vi "CRYO_MASTER_FULL_RUN2.vi"() -> ()   [LabVIEW 2017] (continued)
  T23 = typedef "imagedata.ctl" = cluster{"image type":i32, "image depth":i32, "image":u8[], "mask":u8[], "colors":u32[], "Rectangle":cluster{"left":i16, "top":i16, "right":i16, "bottom":i16}}
  T24 = enum16{"open", "replace", "create", "open or create", "replace or create", "replace or create with confirmation"}
  T25 = cluster{"TimeArray":timestamp[], "DataArrayConv":dbl[]}[]
  T26 = cluster{"IndexArray":i64[], "TimeArray":timestamp[], "DataArrayRaw":dbl[][], "DataArrayConv":dbl[][], "LDArray":dbl[]}
  T27 = cluster{"InstName":string, "Active?":bool, "Status":enum16{"Intialized", "Ready", "Measuring", "Terminated"}, "Labels":string[], "LabelLD":string, "FileFormat":string[], "FileFormatLD":string, "ReadLeakDet?":bool}
  T28 = cluster{"AOUT Labels[0]":string, "AOUT Labels[1]":string, "AOUT Labels[2]":string, "AOUT Labels[3]":string, "AOUT Labels[4]":string, "AOUT Labels[5]":string, "AOUT Labels[6]":string, "AOUT Labels[7]":string, "AOUT Labels[8]":string}
  T29 = cluster{"TimeArray":timestamp[], "DataArrayConv":dbl[]}
  T30 = cluster{"TimeArray":timestamp[], "DataArrayConv (USB6218)":dbl[]}
  T31 = cluster{"TimeArray":timestamp[], "M.A. Array":dbl[]}
  T32 = cluster{"TimeArray":timestamp[], "M.A. Array":dbl[]}[]
  T33 = cluster{"TimeArray":timestamp[], "DataArray":dbl[]}
  T34 = enum16{"USB6210", "USB6218AI", "USB6218AO", "LSI218", "LSI336", "DMMs"}
diagram:
  w15 = TRUE ("create if not found? (T)")
  w19 = errorcluster {"status"=FALSE, "code"=0, "source"=""} ("error in (no error)")
  w4 = errorcluster {"status"=FALSE, "code"=0, "source"=""} ("error in (no error)")
  n1 = while {
    shift-right: [w42] -> _
    shift-left: dbl[] [] -> [w48]
    shift-right: [w45] -> _
    shift-left: timestamp[] [] -> [w47]
    i -> [w46]
    stop <- w49 stop-if-true
    n2 = Wait (ms)(milliseconds to wait=u32 225) -> ()  [unwired: 1 out]
    n3 = event shown="[6] \"OUTPUT (PWR)\", \"OUTPUT (PMC)\": Value Change" {
      selector: _ -> [_ _ _ _ _ _ _]
      dyn-events: _ -> [_ _ _ _ _ _ _]
      timeout: _ -> [_ _ _ _ _ _ _]
      tunnel: [_ TRUE _ _ _ _ _] -> w49
      tunnel: w46 -> [_ _ _ _ w130 _ _]
      tunnel: [_ _ _ _ w129 w213 _] -> w42
      tunnel: w48 -> [_ _ _ _ w126 w213 _]
      tunnel: [w51 w61 _ _ w128 w212 w216] -> w45
      tunnel: w47 -> [w51 w61 _ _ w127 w212 w216]
      tunnel: w46 -> [_ _ w67 w91 _ _ w217]
      tunnel: [_ _ _ _ w117 _ _] -> w41
      event Timeout {
        n4 = event-data() -> ()  [unwired: 1 in, 3 out]
      }
      event "Stop Button": Value Change {
        w52 = FALSE
        n5 = event-data() -> ()  [unwired: 1 in, 3 out]
        n6 = local read "error out (USB6210/6218 DOUT)"() -> (w60:errorcluster)
        n7 = local read "error out (USB6210/6218 AOUT)"() -> (w57:errorcluster)
        n8 = local read "DOUT task out"() -> (w56:refnum<k21>)
        n9 = local read "AO task out"() -> (w63:refnum<k21>)
        n10 = property on="OUTPUT\n(PWR)" class="Bool (strict)"("Value"=w52) -> ()  [unwired: 2 in, 2 out]
        n11 = property on="V2 (N.C.)" class="Bool (strict)"("Val(Sgnl)"=w52) -> ()  [unwired: 2 in, 2 out]
        n12 = property on="OUTPUT\n(PMC)" class="Bool (strict)"("Value"=w52) -> ()  [unwired: 2 in, 2 out]
        n13 = Build Array(w52, w52, w52, w52) -> (w59:bool[])
        n14 = Not(x=w52) -> (.not. x?=w53:bool)
        n15 = call <vilib>:"DAQmx Clear Task.vi"("task in"=w63, "error in"=w57) -> ("error out"=w62:errorcluster)  [unwired: 13 in]
        n16 = property on="V1 (N.O.)" class="Bool (strict)"("Val(Sgnl)"=w53) -> ()  [unwired: 2 in, 2 out]
        n17 = call <vilib>:"DAQmx Write (Digital 1D Bool NChan 1Samp 1Line).vi"("task/channels in"=w56, "data"=w59, "timeout"=10.0, "error in"=w60) -> ("task out"=w55:refnum<k21>, "error out"=w54:errorcluster)  [unwired: 9 in, 1 out]
        n18 = call <vilib>:"DAQmx Clear Task.vi"("task in"=w55, "error in"=w54) -> ("error out"=w64:errorcluster)  [unwired: 13 in]
        n19 = local write "error out (USB6210/6218 AOUT)"(w62) -> ()
        n20 = local write "error out (USB6210/6218 DOUT)"(w64) -> ()
      }
      event "V1 (N.O.)": Value Change {
        n21 = event-data() -> ()  [unwired: 1 in, 3 out]
        n22 = local read "Cycle #"() -> (w70:u32)
        n23 = Greater?(x=w70, y=u32 0) -> (0:w68:bool)
        n24 = case shown="True" w68 {
          tunnel: "V1 (N.O.)" -> [_ w84]
          tunnel: w67 -> [_ w79]
          frame False {
          }
          frame True {
            n25 = Not(x=w84) -> (.not. x?=w86:bool)
            n26 = property on="OUTPUT\n(PMC)" class="Bool (strict)"() -> ("Value"=w71:bool)  [unwired: 2 in, 2 out]
            n27 = local read "error out (USB6210/6218 DOUT)"() -> (w85:errorcluster)
            n28 = property on="OUTPUT\n(PWR)" class="Bool (strict)"() -> ("Value"=w82:bool)  [unwired: 2 in, 2 out]
            n29 = property on="V2 (N.C.)" class="Bool (strict)"() -> ("Value"=w83:bool)  [unwired: 2 in, 2 out]
            n30 = local read "DOUT task out"() -> (w89:refnum<k21>)
            n31 = Build Array(w86, w83, w82, w71) -> (w75:bool[])
            n32 = local read "File Refn USB DO"() -> (w80:refnum<file>)
            n33 = Boolean To (0,1)(Boolean=w75) -> (0, 1=w74:i16[])
            n34 = Initialize Array("%d" ("element"), 3 ("dimension size")) -> (w78:string[])
            n35 = call <vilib>:"DAQmx Write (Digital 1D Bool NChan 1Samp 1Line).vi"("task/channels in"=w89, "data"=w75, "timeout"=10.0, "error in"=w85) -> ("task out"=w87:refnum<k21>, "error out"=w73:errorcluster)  [unwired: 9 in, 1 out]
            n36 = local write "DOUT task out"(w87) -> ()
            n37 = Get Date/Time In Seconds() -> (seconds since 1Jan1904=w81:timestamp)
            n38 = call "FileWrite.vi"("DataArray"=w74, "Time Stamp"=w81, "Error In"=w73, "FileFormat"=w78, "Index"=w79, "refnum in"=w80) -> ("Error Out"=w72:errorcluster)  [unwired: 4 in, 1 out]
            n39 = local write "error out (USB6210/6218 DOUT)"(w72) -> ()
          }
        }
        "V1" <- "V1 (N.O.)"
      }
      event "V2 (N.C.)": Value Change {
        n40 = event-data() -> ()  [unwired: 1 in, 3 out]
        n41 = local read "Cycle #"() -> (w94:u32)
        n42 = Greater?(x=w94, y=u32 0) -> (0:w92:bool)
        n43 = case shown="True" w92 {
          tunnel: "V2 (N.C.)" -> [_ w109]
          tunnel: w91 -> [_ w101]
          frame False {
          }
          frame True {
            n44 = property on="OUTPUT\n(PMC)" class="Bool (strict)"() -> ("Value"=w95:bool)  [unwired: 2 in, 2 out]
            n45 = property on="V1 (N.O.)" class="Bool (strict)"() -> ("Value"=w108:bool)  [unwired: 2 in, 2 out]
            n46 = Not(x=w108) -> (.not. x?=w107:bool)
            n47 = local read "error out (USB6210/6218 DOUT)"() -> (w112:errorcluster)
            n48 = property on="OUTPUT\n(PWR)" class="Bool (strict)"() -> ("Value"=w106:bool)  [unwired: 2 in, 2 out]
            n49 = local read "DOUT task out"() -> (w113:refnum<k21>)
            n50 = Build Array(w107, w109, w106, w95) -> (w104:bool[])
            n51 = local read "File Refn USB DO"() -> (w105:refnum<file>)
            n52 = Boolean To (0,1)(Boolean=w104) -> (0, 1=w103:i16[])
            n53 = Initialize Array("%d" ("element"), 3 ("dimension size")) -> (w98:string[])
            n54 = call <vilib>:"DAQmx Write (Digital 1D Bool NChan 1Samp 1Line).vi"("task/channels in"=w113, "data"=w104, "timeout"=10.0, "error in"=w112) -> ("task out"=w110:refnum<k21>, "error out"=w97:errorcluster)  [unwired: 9 in, 1 out]
            n55 = local write "DOUT task out"(w110) -> ()
            n56 = Get Date/Time In Seconds() -> (seconds since 1Jan1904=w102:timestamp)
            n57 = call "FileWrite.vi"("DataArray"=w103, "Time Stamp"=w102, "Error In"=w97, "FileFormat"=w98, "Index"=w101, "refnum in"=w105) -> ("Error Out"=w96:errorcluster)  [unwired: 4 in, 1 out]
            n58 = local write "error out (USB6210/6218 DOUT)"(w96) -> ()
          }
        }
        "V2" <- "V2 (N.C.)"
      }
      event "Set Current (mA)\n (PMC)", "Set Current (mA)\n (PWR)", "update current": Value Change {
        n59 = event-data() -> ()  [unwired: 1 in, 3 out]
        n60 = case shown="True" "CONTROL KIKUSUI?" {
          tunnel: w130 -> [_ w181]
          tunnel: [w140 w174] -> w129
          tunnel: [w143 w173] -> w128
          tunnel: w127 -> [w145 w176]
          tunnel: w126 -> [w141 w175]
          tunnel: "Set Current (mA)\n (PWR)" -> [_ w153]
          tunnel: "Set Current (mA)\n (PMC)" -> [_ w157]
          frame False {
            w142 = 0.0 ("element")
            n61 = Get Date/Time In Seconds() -> (seconds since 1Jan1904=w144:timestamp)
            n62 = local read "AO task out"() -> (w150:refnum<k21>)
            n63 = Build Array (concatenate)(w145, w144) -> (w143:timestamp[])
            n64 = Build Array (concatenate)(w141, w142) -> (w140:dbl[])
            n65 = Build Array(w142, w142) -> (w148:dbl[])
            n66 = call <vilib>:"DAQmx Write (Analog 1D DBL NChan 1Samp).vi"("task/channels in"=w150, "data"=w148, "timeout"=100.0, "error in"=errorcluster {"status"=FALSE, "code"=0, "source"=""}) -> ("task out"=w151:refnum<k21>, "error out"=w146:errorcluster)  [unwired: 9 in, 1 out]
            n67 = local write "AO task out"(w151) -> ()
            n68 = local write "error out (KIKUSI CTRL)"(w146) -> ()
          }
          frame True {
            w168 = 2 ("index")
            n69 = xnode "Formula"("X1"=w153) -> ("Result"=w170:dbl)  [unwired: 1 in, 1 out]
            n70 = xnode "Formula"("X1"=w157) -> ("Result"=w164:dbl)  [unwired: 1 in, 1 out]
            n71 = Build Array (concatenate)(w175, w153) -> (w174:dbl[])
            n72 = In Range and Coerce(upper limit=10.0, x=w170, lower limit=0.0 ("y")) -> (coerced(x)=w162:dbl, In Range?=w163:bool)
            n73 = In Range and Coerce(upper limit=10.0, x=w164, lower limit=0.0 ("y")) -> (coerced(x)=w159:dbl, In Range?=w160:bool)
            n74 = case shown="False" w163 {
              tunnel: w162 -> [_ w193]
              tunnel: [0.0 ("upper limit") w193] -> w161
              frame False {
              }
              frame True {
              }
            }
            n75 = case shown="True" w160 {
              tunnel: w159 -> [_ w191]
              tunnel: [0.0 ("upper limit") w191] -> w158
              frame False {
              }
              frame True {
              }
            }
            n76 = Multiply(x=w153, y=0.001) -> (x*y=w152:dbl)
            n77 = Multiply(x=w157, y=0.001) -> (x*y=w156:dbl)
            n78 = local read "File Refn USB AO"() -> (w182:refnum<file>)
            n79 = Build Array(w152, w156, w161, w158) -> (w169:dbl[])
            "USB 6218 AOUT" <- w169
            n80 = Initialize Array("%.3f", 4 ("dimension size")) -> (w183:string[])
            n81 = Get Date/Time In Seconds() -> (seconds since 1Jan1904=w177:timestamp)
            n82 = local read "AO task out"() -> (w187:refnum<k21>)
            n83 = call "FileWrite.vi"("DataArray"=w169, "Time Stamp"=w177, "Error In"=errorcluster {"status"=FALSE, "code"=0, "source"=""} ("error in"), "FileFormat"=w183, "Index"=w181, "refnum in"=w182) -> ("Error Out"=w179:errorcluster, "Byte Stream File Refnum"=w178:refnum<file>)  [unwired: 4 in]
            n84 = Build Array (concatenate)(w176, w177) -> (w173:timestamp[])
            n85 = Array Subset(array=w169, index=w168, length=w168) -> (w167:dbl[])
            n86 = local write "File Refn USB AO"(w178) -> ()
            n87 = call <vilib>:"DAQmx Write (Analog 1D DBL NChan 1Samp).vi"("task/channels in"=w187, "data"=w167, "timeout"=100.0, "error in"=w179) -> ("task out"=w188:refnum<k21>, "error out"=→"error out (KIKUSI CTRL)":errorcluster)  [unwired: 9 in, 1 out]
            n88 = local write "AO task out"(w188) -> ()
          }
        }
        n89 = local read "All Labels (USB6218)"() -> (w123:string[])
        n90 = local read "DataArrayConv (USB6218)"() -> (w122:dbl[][])
        n91 = local read "Last Data \n(USB6218)"() -> (w119:dbl[])
        n92 = local read "TimeArray (USB6218)"() -> (w120:timestamp[])
        n93 = Search 1D Array(1D array=w123, element="I_CV") -> (index of element=w124:i32)  [unwired: 1 in]
        n94 = Index Array(array=w122, index (row)=w124) -> (element=w121:dbl[])  [unwired: 1 in]
        n95 = Index Array(array=w119, index=w124) -> (element=w116:dbl)
        n96 = Bundle("TimeArray (USB6218)"=w120, "DataArrayConv (USB6218)"=w121) -> (w117:T19)  [unwired: 1 in]
        n97 = xnode "Formula"("X1"=w116) -> ("Result"=→"Monitor Current (mA)":dbl)  [unwired: 1 in, 1 out]
      }
      event "upper limit (mA)\n (PWR)", "lower limit (mA) \n(PWR)": Value Change {
        n98 = event-data() -> ()  [unwired: 1 in, 6 out]
        n99 = property on="Set Current (mA)\n (PWR)" class="DigNum (strict)"("Maximum"="upper limit (mA)\n (PWR)", "Minimum"="lower limit (mA) \n(PWR)") -> ()  [unwired: 2 in, 2 out]
        n100 = property on="Set Current (mA)\n (PMC)" class="DigNum (strict)"("Maximum"="upper limit (mA)\n (PMC)", "Minimum"="lower limit (mA) \n(PMC)") -> ()  [unwired: 2 in, 2 out]
      }
      event "OUTPUT\n(PWR)", "OUTPUT\n(PMC)": Value Change {
        n101 = event-data() -> ()  [unwired: 1 in, 6 out]
        n102 = local read "Cycle #"() -> (w220:u32)
        n103 = Greater?(x=w220, y=u32 0) -> (0:w218:bool)
        n104 = case shown="True" w218 {
          tunnel: w217 -> [_ w225]
          frame False {
          }
          frame True {
            n105 = property on="V1 (N.O.)" class="Bool (strict)"() -> ("Value"=w236:bool)  [unwired: 2 in, 2 out]
            n106 = Not(x=w236) -> (.not. x?=w235:bool)
            n107 = local read "error out (USB6210/6218 DOUT)"() -> (w239:errorcluster)
            n108 = property on="V2 (N.C.)" class="Bool (strict)"() -> ("Value"=w234:bool)  [unwired: 2 in, 2 out]
            n109 = local read "DOUT task out"() -> (w240:refnum<k21>)
            n110 = Build Array(w235, w234, "OUTPUT\n(PWR)", "OUTPUT\n(PMC)") -> (w223:bool[])
            n111 = local read "File Refn USB DO"() -> (w226:refnum<file>)
            n112 = Boolean To (0,1)(Boolean=w223) -> (0, 1=w222:i16[])
            n113 = call <vilib>:"DAQmx Write (Digital 1D Bool NChan 1Samp 1Line).vi"("task/channels in"=w240, "data"=w223, "timeout"=10.0, "error in"=w239) -> ("task out"=w237:refnum<k21>, "error out"=w230:errorcluster)  [unwired: 9 in, 1 out]
            n114 = Initialize Array("%d" ("element"), 3 ("dimension size")) -> (w228:string[])
            n115 = local write "DOUT task out"(w237) -> ()
            n116 = Get Date/Time In Seconds() -> (seconds since 1Jan1904=w227:timestamp)
            n117 = call "FileWrite.vi"("DataArray"=w222, "Time Stamp"=w227, "Error In"=w230, "FileFormat"=w228, "Index"=w225, "refnum in"=w226) -> ("Error Out"=w229:errorcluster, "Byte Stream File Refnum"=w224:refnum<file>)  [unwired: 4 in]
            n118 = local write "File Refn USB DO"(w224) -> ()
            n119 = local write "error out (USB6210/6218 DOUT)"(w229) -> ()
          }
        }
      }
    }
    n120 = Bundle(w45, w42) -> (w44:cluster{timestamp[], dbl[]})  [unwired: 1 in]
    n121 = Build Array(w44, w41) -> (→"Graph 7":T10)
  }
  n122 = while {
    shift-right: [w249] -> _
    shift-left: refnum<class "6240AData.lvclass"> refnum ("6240AData.lvclass") -> [w247]
    shift-right: [w245] -> _
    shift-left: errorcluster {"status"=FALSE, "code"=0, "source"=""} ("error in (no error)") -> [w246]
    i -> [w241]
    stop <- w248 stop-if-true
    n123 = Wait (ms)(milliseconds to wait=u32 231) -> ()  [unwired: 1 out]
    n124 = Equal?(x=w241, y=0) -> (x = y?=w243:bool)
    n125 = case shown="True" w243 {
      frame False {
      }
      frame True {
        n126 = property on="Initialized?" class="Bool (strict)"("Val(Sgnl)"=FALSE ("Value (Signaling)")) -> ()  [unwired: 2 in, 2 out]
      }
    }
    n127 = event shown="[2] \"upper limit (mA)\", \"lower limit (mA)\": Value Change" {
      selector: _ -> [_ _ _ _ _]
      dyn-events: _ -> [_ _ _ _ _]
      timeout: _ -> [_ _ _ _ _]
      tunnel: [w252 w267 _ w316 w337] -> w249
      tunnel: [_ _ _ _ TRUE ("Value (Signaling)")] -> w248
      tunnel: w247 -> [w252 w266 _ w300 w335]
      tunnel: w246 -> [w251 w265 _ w299 w333]
      tunnel: [w251 w264 _ w314 w336] -> w245
      tunnel: w241 -> [_ w263 _ _ _]
      tunnel: w241 -> [_ _ _ w308 _]
      event Timeout {
        n128 = event-data() -> ()  [unwired: 1 in, 3 out]
      }
      event "update values", "SetCurrent 1 (mA)", "SetCurrent 2 (mA)": Value Change {
        w256 = 1000.0 ("y")
        n129 = event-data() -> ()  [unwired: 1 in, 6 out]
        n130 = local read "Initialized?"() -> (w262:bool)
        n131 = Divide(x="SetCurrent 1 (mA)", y=w256) -> (x/y=w257:dbl)
        n132 = Divide(x="SetCurrent 2 (mA)", y=w256) -> (x/y=w258:dbl)
        n133 = Build Array(w257, w258) -> (w255:dbl[])
        n134 = Not Equal?(x=w262, y=FALSE) -> (x != y?=w260:bool)
        n135 = case shown="True" w260 {
          tunnel: [w269 w293] -> w267
          tunnel: "Output\n (ADCMT)" -> [_ w292]
          tunnel: w266 -> [w269 w291]
          tunnel: w265 -> [w268 w290]
          tunnel: [w268 w289] -> w264
          tunnel: w263 -> [_ w285]
          tunnel: w255 -> [_ w271]
          frame False {
          }
          frame True {
            w278 = 1 ("index (col)")
            w279 = 0 ("disabled index (col)")
            n136 = call-dynamic "6240AData_execute.vi"("6240AData in"=w291, "SetCurrent (A)"=w271, "FileFormat"="%3.5f", "Output status"=w292, "ExecutionIndex"=w285, "error in (no error)"=w290) -> ("ActualVoltage (V)"=w270:dbl[], "ActualCurrent (A)"=w284:dbl[], "6240AData out"=w293:refnum<class "6240AData.lvclass">, "appended array"=w274:timestamp[], "SetCurrentArray"=w280:dbl[][], "ActualCurrentArray"=w287:dbl[][], "error out"=w289:errorcluster)  [unwired: 3 in]
            n137 = property on="ActualVoltage (V)" class="Arr (strict)"("Val(Sgnl)"=w270) -> ()  [unwired: 2 in, 2 out]
            n138 = property on="ActualCurrent (A)" class="Arr (strict)"("Val(Sgnl)"=w284) -> ()  [unwired: 2 in, 2 out]
            n139 = Index Array(array=w287, index (col) #1=w279, index (col) #2=w278) -> (element #1=w288:dbl[], element #2=w282:dbl[])  [unwired: 2 in]
            n140 = Index Array(array=w280, index (col) #1=w279, index (col) #2=w278) -> (element #1=w276:dbl[], element #2=w273:dbl[])  [unwired: 2 in]
            n141 = Bundle("appended array"=w274, "ActualCurrentArray"=w288) -> (w283:T20)  [unwired: 1 in]
            n142 = Bundle("appended array"=w274, "ActualCurrentArray"=w282) -> (w277:T20)  [unwired: 1 in]
            n143 = Bundle("appended array"=w274, "SetCurrentArray"=w276) -> (w275:T21)  [unwired: 1 in]
            n144 = Bundle("appended array"=w274, "SetCurrentArray"=w273) -> (w272:T21)  [unwired: 1 in]
            n145 = Build Array(w283, w277, w275, w272) -> (→"Graph 6":T22)
          }
        }
      }
      event "upper limit (mA)", "lower limit (mA)": Value Change {
        n146 = event-data() -> ()  [unwired: 1 in, 6 out]
        n147 = property on="SetCurrent 1 (mA)" class="DigNum (strict)"("Maximum"="upper limit (mA)", "Minimum"="lower limit (mA)") -> ()  [unwired: 2 in, 2 out]
        n148 = property on="SetCurrent 2 (mA)" class="DigNum (strict)"("Maximum"="upper limit (mA)", "Minimum"="lower limit (mA)") -> ()  [unwired: 2 in, 2 out]
      }
      event "Initialize": Value Change {
        w310 = FALSE
        n149 = event-data() -> ()  [unwired: 1 in, 6 out]
        n150 = local read "Initialized?"() -> (w298:bool)
        n151 = case shown="True" w298 {
          tunnel: w300 -> [w326 w330]
          tunnel: w299 -> [w325 w329]
          tunnel: [w326 w328] -> w297
          tunnel: [w325 w327] -> w296
          frame False {
          }
          frame True {
            n152 = call-dynamic "6240AData_terrminate.vi"("error in (no error)"=w329, "6240AData in"=w330) -> ("error out"=w327:errorcluster, "6240AData out"=w328:refnum<class "6240AData.lvclass">)  [unwired: 8 in]
          }
        }
        n153 = property on="Initialized?" class="Bool (strict)"("Val(Sgnl)"=TRUE ("Value (Signaling)")) -> ()  [unwired: 2 in, 2 out]
        n154 = local read "SetCurrent 2 (mA)"() -> (w303:dbl)
        n155 = local read "SetCurrent 1 (mA)"() -> (w306:dbl)
        n156 = local read "RUN Identifier"() -> (w318:string)
        n157 = local read "Base Path"() -> (w319:path)
        n158 = Divide(x=w306, y=1000.0) -> (x/y=w305:dbl)
        n159 = Divide(x=w303, y=1000.0) -> (x/y=w302:dbl)
        n160 = Get Date/Time In Seconds() -> ()  [unwired: 1 out]
        n161 = call-dynamic "6240AData_initialize.vi"("6240AData in"=w297, "RunIdentifier"=w318, "InstName"="InstName", "base path"=w319, "VISA"="VISA", "error in (no error)"=w296, "CtrlLabels"="CtrlLabels", "Voltage limits (V)"="Voltage limits (V)") -> ("6240AData out"=w317:refnum<class "6240AData.lvclass">, "error out"=w315:errorcluster)  [unwired: 6 in]
        n162 = Build Array(w305, w302) -> (w301:dbl[])
        n163 = Build Array(w310, w310) -> (w309:bool[])
        n164 = call-dynamic "6240AData_execute.vi"("6240AData in"=w317, "SetCurrent (A)"=w301, "FileFormat"="%3.5f", "Output status"=w309, "ExecutionIndex"=w308, "error in (no error)"=w315) -> ("ActualVoltage (V)"=w312:dbl[], "ActualCurrent (A)"=w311:dbl[], "6240AData out"=w316:refnum<class "6240AData.lvclass">, "error out"=w314:errorcluster)  [unwired: 3 in, 3 out]
        n165 = property on="ActualVoltage (V)" class="Arr (strict)"("Val(Sgnl)"=w312) -> ()  [unwired: 2 in, 2 out]
        n166 = property on="ActualCurrent (A)" class="Arr (strict)"("Val(Sgnl)"=w311) -> ()  [unwired: 2 in, 2 out]
      }
      event "Stop Button": Value Change {
        n167 = event-data() -> ()  [unwired: 1 in, 6 out]
        n168 = local read "Initialized?"() -> (w331:bool)
        n169 = case shown="False" w331 {
          tunnel: w335 -> [w340 w352]
          tunnel: [w340 w351] -> w334
          tunnel: w333 -> [w339 w350]
          tunnel: [w339 w349] -> w332
          frame False {
          }
          frame True {
            w356 = FALSE
            n170 = local read "SetCurrent 2 (mA)"() -> (w342:dbl)
            n171 = local read "SetCurrent 1 (mA)"() -> (w346:dbl)
            n172 = Divide(x=w346, y=1000.0) -> (x/y=w344:dbl)
            n173 = Divide(x=w342, y=1000.0) -> (x/y=w341:dbl)
            n174 = Build Array(w344, w341) -> (w348:dbl[])
            n175 = Build Array(w356, w356) -> (w347:bool[])
            n176 = property on="Output\n (ADCMT)" class="Arr (strict)"("Val(Sgnl)"=w347) -> ()  [unwired: 2 in, 2 out]
            n177 = call-dynamic "6240AData_execute.vi"("6240AData in"=w352, "SetCurrent (A)"=w348, "FileFormat"="%3.5f", "Output status"=w347, "error in (no error)"=w350) -> ("ActualVoltage (V)"=w353:dbl[], "ActualCurrent (A)"=w354:dbl[], "6240AData out"=w351:refnum<class "6240AData.lvclass">, "error out"=w349:errorcluster)  [unwired: 4 in, 3 out]
            n178 = property on="ActualVoltage (V)" class="Arr (strict)"("Val(Sgnl)"=w353) -> ()  [unwired: 2 in, 2 out]
            n179 = property on="ActualCurrent (A)" class="Arr (strict)"("Val(Sgnl)"=w354) -> ()  [unwired: 2 in, 2 out]
          }
        }
        n180 = call-dynamic "6240AData_terrminate.vi"("error in (no error)"=w332, "6240AData in"=w334) -> ("error out"=w336:errorcluster, "6240AData out"=w337:refnum<class "6240AData.lvclass">)  [unwired: 8 in]
      }
    }
    "error out (ADCMT6420A)" <- w245
  }
  n181 = while {
    stop <- w365 stop-if-true
    n182 = Get Date/Time In Seconds() -> (seconds since 1Jan1904=w364:timestamp)
    n183 = Format Date/Time String(time format string (%c)="%Y%m", seconds (now)=w364) -> (date/time string=w361:string)  [unwired: 1 in]
    n184 = Build Path(base path="Base Path (screenshots)", name or relative path=w361) -> (appended path=w360:path)
    n185 = Create Folder(path (use dialog)=w360, error in=errorcluster {"status"=FALSE, "code"=0, "source"=""}) -> (created path=w357:path, error out=→"error out (monthly folder creation)":errorcluster)  [unwired: 1 in, 1 out]
    n186 = event shown="[1] \"Frontpanel screenshots\": Value Change" {
      selector: _ -> [_ _ _]
      dyn-events: _ -> [_ _ _]
      timeout: _ -> [_ _ _]
      tunnel: [FALSE _ TRUE] -> w365
      tunnel: w357 -> [_ w373 _]
      tunnel: w364 -> [_ w372 _]
      event Timeout {
        n187 = event-data() -> ()  [unwired: 1 in, 3 out]
      }
      event "Frontpanel screenshots": Value Change {
        n188 = event-data() -> ()  [unwired: 1 in, 3 out]
        n189 = property class="TabCtl (strict)"() -> ("Value"=w370:T1)  [unwired: 2 in, 2 out]
        n190 = stacked-sequence {
          tunnel: w373 -> [w379 w401 w423 w445 w467 w489 w511 w533 w555 _]
          tunnel: w372 -> [w378 w400 w422 w444 w466 w488 w510 w532 w554 _]
          tunnel: [w376 _ _ _ _ _ _ _ _ _] -> w371
          tunnel: w370 -> [w375 _ _ _ _ _ _ _ _ _]
          tunnel: [w375 _ _ _ _ _ _ _ _ _] -> w369
          tunnel: "cryostatus_" ("string") -> [w374 w397 w419 w441 w463 w485 w507 w529 w551 _]
          frame #0 {
            n191 = flat-sequence {
              tunnel: w378 -> [w381]
              tunnel: [w381] -> w377
              tunnel: w379 -> [w396]
              tunnel: w377 -> [w384]
              tunnel: [w383] -> w376
              tunnel: w374 -> [w382]
              frame #0 {
                n192 = property class="TabCtl (strict)"("Val(Sgnl)"=T1."NI USB CONFIG" ("Value (Signaling)")) -> ()  [unwired: 2 in, 2 out]
              }
              frame #1 {
                w394 = "_" ("string")
                n193 = local read "Cycle #"() -> (w392:u32)
                n194 = call "LV_UNIXTIME.vi"("current time"=w384) -> ("date/time string"=w395:string)  [unwired: 9 in, 1 out]
                n195 = Format Value(format string="%06d", value (0)=w392) -> (output string=w391:string)  [unwired: 1 in]
                n196 = Concatenate Strings(w382, w395, w394, w391, w394, "page1.png" ("string")) -> (w389:string)
                n197 = invoke class="TabCtl (strict)" method="Get Image"(error in=errorcluster {"status"=FALSE, "code"=0, "source"=""} ("error in (no error)")) -> (error out=w385:errorcluster, "image data"=w387:T23)  [unwired: 5 in, 4 out]
                n198 = Build Path(base path=w396, name or relative path=w389) -> (appended path=w388:path)
                n199 = call <vilib>:"Write PNG File.vi"("error in (no error)"=w385, "image data"=w387, "path to PNG file"=w388) -> ("error out"=w383:errorcluster)  [unwired: 7 in, 1 out]
              }
            }
          }
          frame #1 {
            n200 = flat-sequence {
              tunnel: w400 -> [w403]
              tunnel: [w403] -> w399
              tunnel: w401 -> [w418]
              tunnel: w399 -> [w406]
              tunnel: [w405] -> w398
              tunnel: w397 -> [w404]
              frame #0 {
                n201 = property class="TabCtl (strict)"("Val(Sgnl)"=T1."LSI CONFIG" ("Value (Signaling)")) -> ()  [unwired: 2 in, 2 out]
              }
              frame #1 {
                w416 = "_" ("string")
                n202 = local read "Cycle #"() -> (w414:u32)
                n203 = call "LV_UNIXTIME.vi"("current time"=w406) -> ("date/time string"=w417:string)  [unwired: 9 in, 1 out]
                n204 = Format Value(format string="%06d", value (0)=w414) -> (output string=w413:string)  [unwired: 1 in]
                n205 = Concatenate Strings(w404, w417, w416, w413, w416, "page2.png" ("string")) -> (w411:string)
                n206 = invoke class="TabCtl (strict)" method="Get Image"(error in=errorcluster {"status"=FALSE, "code"=0, "source"=""} ("error in (no error)")) -> (error out=w407:errorcluster, "image data"=w409:T23)  [unwired: 5 in, 4 out]
                n207 = Build Path(base path=w418, name or relative path=w411) -> (appended path=w410:path)
                n208 = call <vilib>:"Write PNG File.vi"("error in (no error)"=w407, "image data"=w409, "path to PNG file"=w410) -> ("error out"=w405:errorcluster)  [unwired: 7 in, 1 out]
              }
            }
            n209 = local write "error out (frontpanel screenshots)"(w398) -> ()
          }
          frame #2 {
            n210 = flat-sequence {
              tunnel: w422 -> [w425]
              tunnel: [w425] -> w421
              tunnel: w423 -> [w440]
              tunnel: w421 -> [w428]
              tunnel: [w427] -> w420
              tunnel: w419 -> [w426]
              frame #0 {
                n211 = property class="TabCtl (strict)"("Val(Sgnl)"=T1."MEASUREMENT" ("Value (Signaling)")) -> ()  [unwired: 2 in, 2 out]
              }
              frame #1 {
                w438 = "_" ("string")
                n212 = local read "Cycle #"() -> (w436:u32)
                n213 = Format Value(format string="%06d", value (0)=w436) -> (output string=w435:string)  [unwired: 1 in]
                n214 = call "LV_UNIXTIME.vi"("current time"=w428) -> ("date/time string"=w439:string)  [unwired: 9 in, 1 out]
                n215 = Concatenate Strings(w426, w439, w438, w435, w438, "page3.png" ("string")) -> (w433:string)
                n216 = invoke class="TabCtl (strict)" method="Get Image"(error in=errorcluster {"status"=FALSE, "code"=0, "source"=""} ("error in (no error)")) -> (error out=w429:errorcluster, "image data"=w431:T23)  [unwired: 5 in, 4 out]
                n217 = Build Path(base path=w440, name or relative path=w433) -> (appended path=w432:path)
                n218 = call <vilib>:"Write PNG File.vi"("error in (no error)"=w429, "image data"=w431, "path to PNG file"=w432) -> ("error out"=w427:errorcluster)  [unwired: 7 in, 1 out]
              }
            }
            n219 = local write "error out (frontpanel screenshots)"(w420) -> ()
          }
          frame #3 {
            n220 = flat-sequence {
              tunnel: w444 -> [w447]
              tunnel: [w447] -> w443
              tunnel: w445 -> [w462]
              tunnel: w443 -> [w450]
              tunnel: [w449] -> w442
              tunnel: w441 -> [w448]
              frame #0 {
                n221 = property class="TabCtl (strict)"("Val(Sgnl)"=T1."HE AUTO FILL" ("Value (Signaling)")) -> ()  [unwired: 2 in, 2 out]
              }
              frame #1 {
                w460 = "_" ("string")
                n222 = local read "Cycle #"() -> (w458:u32)
                n223 = Format Value(format string="%06d", value (0)=w458) -> (output string=w457:string)  [unwired: 1 in]
                n224 = call "LV_UNIXTIME.vi"("current time"=w450) -> ("date/time string"=w461:string)  [unwired: 9 in, 1 out]
                n225 = Concatenate Strings(w448, w461, w460, w457, w460, "page4.png" ("string")) -> (w455:string)
                n226 = invoke class="TabCtl (strict)" method="Get Image"(error in=errorcluster {"status"=FALSE, "code"=0, "source"=""} ("error in (no error)")) -> (error out=w451:errorcluster, "image data"=w453:T23)  [unwired: 5 in, 4 out]
                n227 = Build Path(base path=w462, name or relative path=w455) -> (appended path=w454:path)
                n228 = call <vilib>:"Write PNG File.vi"("error in (no error)"=w451, "image data"=w453, "path to PNG file"=w454) -> ("error out"=w449:errorcluster)  [unwired: 7 in, 1 out]
              }
            }
            n229 = local write "error out (frontpanel screenshots)"(w442) -> ()
          }
          frame #4 {
            n230 = flat-sequence {
              tunnel: w466 -> [w469]
              tunnel: [w469] -> w465
              tunnel: w467 -> [w484]
              tunnel: w465 -> [w472]
              tunnel: [w471] -> w464
              tunnel: w463 -> [w470]
              frame #0 {
                n231 = property class="TabCtl (strict)"("Val(Sgnl)"=T1."VALVE/HEATER CTRL" ("Value (Signaling)")) -> ()  [unwired: 2 in, 2 out]
              }
              frame #1 {
                w482 = "_" ("string")
                n232 = local read "Cycle #"() -> (w480:u32)
                n233 = call "LV_UNIXTIME.vi"("current time"=w472) -> ("date/time string"=w483:string)  [unwired: 9 in, 1 out]
                n234 = Format Value(format string="%06d", value (0)=w480) -> (output string=w479:string)  [unwired: 1 in]
                n235 = Concatenate Strings(w470, w483, w482, w479, w482, "page5.png" ("string")) -> (w477:string)